vi "UHR-Fleezers Control (host) - Avogadro v3.vi"() -> ()   [LabVIEW 2014] (continued)
        n1387 = case shown="True" "Vortran Laser ON" {
          tunnel: "Laser interlacing mode" -> [_ w2246]
          tunnel: [enum32{"Laser ON", "Laser OFF", "Interlace"}."Laser OFF" ("Green laser mode") w2246] -> w2222
          tunnel: [FALSE w2242] -> w2221
          frame False {
          }
          frame True {
            n1388 = local read "Green FB On/Off"() -> (w2243:bool)
            n1389 = Equal?(x=w2246, y=enum32{"Laser ON", "Laser OFF", "Interlace"}."Interlace") -> (x = y?=w2244:bool)
            n1390 = And(x=w2244, y=w2243) -> (x .and. y?=w2242:bool)
          }
        }
        n1391 = case shown="True" "Red Laser ON" {
          tunnel: "Laser interlacing mode" -> [_ w2239]
          tunnel: [enum32{"Laser ON", "Laser OFF", "Interlace"}."Laser OFF" ("Green laser mode") w2239] -> w2218
          tunnel: [FALSE w2235] -> w2217
          frame False {
          }
          frame True {
            n1392 = local read "Red FB On/Off"() -> (w2236:bool)
            n1393 = Equal?(x=w2239, y=enum32{"Laser ON", "Laser OFF", "Interlace"}."Interlace") -> (x = y?=w2237:bool)
            n1394 = And(x=w2237, y=w2236) -> (x .and. y?=w2235:bool)
          }
        }
        n1395 = case shown="True" "Blue Laser ON" {
          tunnel: "Laser interlacing mode" -> [_ w2230]
          tunnel: [enum32{"Laser ON", "Laser OFF", "Interlace"}."Laser OFF" ("Green laser mode") w2230] -> w2214
          tunnel: [FALSE w2228] -> w2213
          frame False {
          }
          frame True {
            n1396 = local read "Blue FB On/Off"() -> (w2229:bool)
            n1397 = Equal?(x=w2230, y=enum32{"Laser ON", "Laser OFF", "Interlace"}."Interlace") -> (x = y?=w2231:bool)
            n1398 = And(x=w2231, y=w2229) -> (x .and. y?=w2228:bool)
          }
        }
        n1399 = xnode "Read/Write Control"("FPGA VI Reference In"=w2212, "Operating Mode"=w2222, "Operating Mode 2"=w2222, "Green FB On/Off"=w2221, "Red Laser Operating Mode"=w2218, "RI Operating Mode 2"=w2218, "Red FB On/Off"=w2217, "BI Operating Mode (AO)"=w2214, "Blue Laser Operating Mode (D)"=w2214, "Blue FB On/Off"=w2213) -> ("error out"=w2223:errorcluster)  [unwired: 1 in, 1 out]
        n1400 = local read "Red FB On/Off"() -> (w2195:bool)
        n1401 = local read "Vortran Laser ON"() -> (w2196:bool)
        n1402 = local read "Green FB On/Off"() -> (w2197:bool)
        n1403 = local read "Red Laser ON"() -> (w2194:bool)
        n1404 = And(x=w2195, y=w2194) -> (x .and. y?=w2200:bool)
        n1405 = And(x=w2197, y=w2196) -> (x .and. y?=w2206:bool)
        n1406 = local read "Red laser intensity (V)"() -> (w2199:dbl)
        n1407 = local read "Red FB Setpoint (mV)"() -> (w2198:dbl)
        n1408 = local read "Green FB Setpoint (mV)"() -> (w2209:dbl)
        n1409 = local read "Green laser intensity (V)"() -> (w2211:dbl)
        n1410 = Multiply(x=w2199, y=1000.0) -> (x*y=w2203:dbl)
        n1411 = Subtract(x=w2198, y=5.0) -> (x-y=w2202:dbl)
        n1412 = Multiply(x=w2211, y=1000.0) -> (x*y=w2208:dbl)
        n1413 = Subtract(x=w2209, y=5.0) -> (x-y=w2207:dbl)
        n1414 = Less Or Equal?(x=w2203, y=w2202) -> (x <= y?=w2201:bool)
        n1415 = Less Or Equal?(x=w2208, y=w2207) -> (x <= y?=w2205:bool)
        n1416 = And(x=w2200, y=w2201) -> (x .and. y?=w2190:bool)
        n1417 = And(x=w2206, y=w2205) -> (x .and. y?=w2191:bool)
        n1418 = Or(x=w2191, y=w2190) -> (x .or. y?=w2189:bool)
        n1419 = case shown="True" w2189 {
          frame False {
            n1420 = local write "Laser Intensity Low (bugs to fix)"(FALSE ("Laser Intensity Low")) -> ()
          }
          frame True {
            n1421 = local write "Laser Intensity Low (bugs to fix)"(TRUE ("Laser Intensity Low")) -> ()
          }
        }
      }
      event "Laser choice 0", "Laser choice 1", "Laser choice 2", "FL interlace ON count 0", "Fl interlace ON count 1", "FL interlace ON count 2", "FL interlace OFF count 0", "FL interlace OFF count 1", "FL interlace OFF count 2": Value Change {
        n1422 = event-data() -> ()  [unwired: 7 out]
        n1423 = xnode "Read/Write Control"("FPGA VI Reference In"=w2247, "FL interlace ON count 0"="FL interlace ON count 0", "Fl interlace ON count 1"="Fl interlace ON count 1", "FL interlace ON count 2"="FL interlace ON count 2", "FL interlace OFF count 0"="FL interlace OFF count 0", "FL interlace OFF count 1"="FL interlace OFF count 1", "FL interlace OFF count 2"="FL interlace OFF count 2", "Laser choice 0"="Laser choice 0", "Laser choice 1"="Laser choice 1", "Laser choice 2"="Laser choice 2") -> ()  [unwired: 1 in, 2 out]
      }
      event "Invert laser interlacing", "RF BD 2 to green AOM": Value Change {
        n1424 = event-data() -> ()  [unwired: 7 out]
        n1425 = local read "RF BD 2 to green AOM"() -> (w2257:bool)
        n1426 = xnode "Read/Write Control"("FPGA VI Reference In"=w2258, "Invert GI"="Invert laser interlacing", "Invert GI 2"="Invert laser interlacing", "Invert RI"="Invert laser interlacing", "Invert RI 2"="Invert laser interlacing", "Invert BI (AO)"="Invert laser interlacing", "Invert BI (D)"="Invert laser interlacing", "RF synth bd controls green"=w2257) -> ("error out"=w2260:errorcluster)  [unwired: 1 in, 1 out]
      }
      event "Green FB Setpoint (mV)", "Green FB Gains", "Green FB On/Off", "Green Intensity % (FB OFF)", "Green int current ON count adj": Value Change {
        n1427 = event-data() -> ()  [unwired: 7 out]
        n1428 = local read "Green FB Setpoint (mV)"() -> (w2280:dbl)
        n1429 = Multiply(x=w2280, y=3.2767) -> (x*y=w2279:dbl)
        n1430 = local read "Green Intensity % (FB OFF)"() -> (w2283:dbl)
        n1431 = Multiply(x=w2283, y=655.35) -> (x*y=w2284:dbl)
        n1432 = To Unsigned Word Integer(number=w2284) -> (unsigned 16bit integer=w2282:u16)
        n1433 = local read "Green int current ON count adj"() -> (w2286:u32)
        n1434 = local read "Laser interlacing mode"() -> (w2277:enum32{"Laser ON", "Laser OFF", "Interlace"})
        n1435 = local read "Green FB Gains"() -> (w2274:T18)
        n1436 = local read "Vortran Laser ON"() -> (w2278:bool)
        n1437 = local read "Green FB On/Off"() -> (w2287:bool)
        n1438 = Equal?(x=w2277, y=enum32{"Laser ON", "Laser OFF", "Interlace"}."Interlace") -> (x = y?=w2275:bool)
        n1439 = Unbundle By Name(w2274) -> ("proportional gain (Kc)"=w2273:i16, "integral gain (Kc*Ts/Ti)"=w2272:i16, "derivative gain (Kc*Td/Ts)"=w2271:i16)
        n1440 = Compound Arithmetic op=AND(w2275, w2287, w2278) -> (w2261:bool)
        n1441 = local read "Green FB Setpoint (mV)"() -> (w2265:dbl)
        n1442 = local read "Green laser intensity (V)"() -> (w2268:dbl)
        n1443 = xnode "Read/Write Control"("FPGA VI Reference In"=w2270, "Green FB Setpoint"=w2279, "Green FB On/Off"=w2261, "Current Out"=w2282, "Green int current ON count adj"=w2286, "P3"=w2273, "I3"=w2272, "D3"=w2271) -> ("error out"=w2288:errorcluster)  [unwired: 1 in, 1 out]
        n1444 = Multiply(x=w2268, y=1000.0) -> (x*y=w2264:dbl)
        n1445 = Subtract(x=w2265, y=5.0) -> (x-y=w2263:dbl)
        n1446 = Less Or Equal?(x=w2264, y=w2263) -> (x <= y?=w2262:bool)
        n1447 = And(x=w2261, y=w2262) -> (x .and. y?=w2269:bool)
        n1448 = case shown="True" w2269 {
          frame False {
            n1449 = local write "Laser Intensity Low (bugs to fix)"(FALSE ("Laser Intensity Low")) -> ()
          }
          frame True {
            n1450 = local write "Laser Intensity Low (bugs to fix)"(TRUE ("Laser Intensity Low")) -> ()
          }
        }
      }
      event "Blue FB Setpoint (mV)", "Blue FB Gains", "Blue FB On/Off", "Blue Intensity % (FB OFF)", "Blue int AO ON count adjust": Value Change {
        # "Triggers blue laser serial command"
        # "16 bit analog out"
        n1451 = event-data() -> ()  [unwired: 7 out]
        n1452 = Multiply(x="Blue FB Setpoint (mV)", y=3.2767) -> (x*y=w2308:dbl)
        n1453 = Multiply(x="Blue Intensity % (FB OFF)", y=0.8) -> (x*y=w2291:dbl)
        n1454 = Number To Decimal String(number=w2291) -> (decimal integer string=w2292:string)  [unwired: 1 in]
        n1455 = Multiply(x="Blue Intensity % (FB OFF)", y=655.35) -> (x*y=w2311:dbl)
        n1456 = local write "Blue Laser Power (mW)\n(Constant Power Mode)"(w2292) -> ()
        n1457 = To Unsigned Word Integer(number=w2311) -> (unsigned 16bit integer=w2310:u16)
        n1458 = local read "Laser interlacing mode"() -> (w2306:enum32{"Laser ON", "Laser OFF", "Interlace"})
        n1459 = Unbundle By Name("Blue FB Gains") -> ("proportional gain (Kc)"=w2303:i16, "integral gain (Kc*Ts/Ti)"=w2302:i16, "derivative gain (Kc*Td/Ts)"=w2301:i16)
        n1460 = local read "Blue Laser ON"() -> (w2296:bool)
        n1461 = Equal?(x=w2306, y=enum32{"Laser ON", "Laser OFF", "Interlace"}."Interlace") -> (x = y?=w2304:bool)
        n1462 = Compound Arithmetic op=AND(w2304, "Blue FB On/Off", w2296) -> (w2307:bool)
        n1463 = xnode "Read/Write Control"("FPGA VI Reference In"=w2295, "Blue FB Setpoint"=w2308, "Blue FB On/Off"=w2307, "BI Current Out"=w2310, "Blue current ON count adj (AO)"="Blue int AO ON count adjust", "P5"=w2303, "I5"=w2302, "D5"=w2301) -> ("error out"=w2313:errorcluster)  [unwired: 1 in, 1 out]
      }
      event "Red FB Setpoint (mV)", "Red FB Gains", "Red FB On/Off", "Red Intensity % (FB OFF)": Value Change {
        n1464 = event-data() -> ()  [unwired: 7 out]
        n1465 = local read "Red FB Setpoint (mV)"() -> (w2334:dbl)
        n1466 = Multiply(x=w2334, y=3.2767) -> (x*y=w2333:dbl)
        n1467 = local read "Red Intensity % (FB OFF)"() -> (w2324:dbl)
        n1468 = Multiply(x=w2324, y=655.35) -> (x*y=w2337:dbl)
        n1469 = To Unsigned Word Integer(number=w2337) -> (unsigned 16bit integer=w2336:u16)
        n1470 = local read "Laser interlacing mode"() -> (w2331:enum32{"Laser ON", "Laser OFF", "Interlace"})
        n1471 = local read "Red FB Gains"() -> (w2328:T18)
        n1472 = local read "Red Laser ON"() -> (w2332:bool)
        n1473 = local read "Red FB On/Off"() -> (w2339:bool)
        n1474 = Equal?(x=w2331, y=enum32{"Laser ON", "Laser OFF", "Interlace"}."Interlace") -> (x = y?=w2329:bool)
        n1475 = Unbundle By Name(w2328) -> ("proportional gain (Kc)"=w2327:i16, "integral gain (Kc*Ts/Ti)"=w2326:i16, "derivative gain (Kc*Td/Ts)"=w2325:i16)
        n1476 = Compound Arithmetic op=AND(w2329, w2339, w2332) -> (w2316:bool)
        n1477 = local read "Red laser intensity (V)"() -> (w2315:dbl)
        n1478 = local read "Red FB Setpoint (mV)"() -> (w2314:dbl)
        n1479 = xnode "Read/Write Control"("FPGA VI Reference In"=w2323, "Red FB Setpoint"=w2333, "Red FB On/Off"=w2316, "RI Current Out"=w2336, "P4"=w2327, "I4"=w2326, "D4"=w2325) -> ("error out"=w2340:errorcluster)  [unwired: 1 in, 1 out]
        n1480 = Multiply(x=w2315, y=1000.0) -> (x*y=w2320:dbl)
        n1481 = Subtract(x=w2314, y=5.0) -> (x-y=w2319:dbl)
        n1482 = Less Or Equal?(x=w2320, y=w2319) -> (x <= y?=w2318:bool)
        n1483 = And(x=w2316, y=w2318) -> (x .and. y?=w2317:bool)
        n1484 = case shown="False" w2317 {
          frame False {
            n1485 = local write "Laser Intensity Low (bugs to fix)"(FALSE ("Laser Intensity Low")) -> ()
          }
          frame True {
            n1486 = local write "Laser Intensity Low (bugs to fix)"(TRUE ("Laser Intensity Low")) -> ()
          }
        }
      }
      event "+ phase (APD 1 Gate)", "- phase (APD 1 Gate)", "+ phase (APD 2 Gate)", "- phase (APD 2 Gate)", "+ phase (APD 3 Gate)", "- phase (APD 3 Gate)", "+ phase (APD Acq)", "- phase (APD Acq)": Value Change {
        n1487 = event-data() -> ()  [unwired: 7 out]
        n1488 = local read "Phase Adj. (APD 1 Gate)"() -> (w2363:i16)
        n1489 = Or(x="- phase (APD 1 Gate)", y="+ phase (APD 1 Gate)") -> (x .or. y?=w2365:bool)
        n1490 = Negate(x=w2363) -> (-x=w2370:i16)
        n1491 = Select(t=w2370, s="+ phase (APD 1 Gate)", f=w2363) -> (s? t:f=w2369:i16)
        n1492 = local read "Phase Adj. (APD 2 Gate)"() -> (w2360:i16)
        n1493 = Or(x="- phase (APD 2 Gate)", y="+ phase (APD 2 Gate)") -> (x .or. y?=w2358:bool)
        n1494 = Negate(x=w2360) -> (-x=w2362:i16)
        n1495 = Select(t=w2362, s="+ phase (APD 2 Gate)", f=w2360) -> (s? t:f=w2359:i16)
        n1496 = Negate(x="Phase Adj. (APD 3 Gate)") -> (-x=w2357:i16)
        n1497 = Or(x="- phase (APD 3 Gate)", y="+ phase (APD 3 Gate)") -> (x .or. y?=w2353:bool)
        n1498 = Select(t=w2357, s="+ phase (APD 3 Gate)", f="Phase Adj. (APD 3 Gate)") -> (s? t:f=w2354:i16)
        n1499 = local read "Phase Adj. (APD Acq)"() -> (w2351:i16)
        n1500 = Or(x="- phase (APD Acq)", y="+ phase (APD Acq)") -> (x .or. y?=w2349:bool)
        n1501 = Negate(x=w2351) -> (-x=w2352:i16)
        n1502 = Select(t=w2352, s="+ phase (APD Acq)", f=w2351) -> (s? t:f=w2350:i16)
        n1503 = xnode "Read/Write Control"("FPGA VI Reference In"=w2343, "Phase count adjustment (APD 1 Gate)"=w2369, "Phase count adjustment (APD 2 Gate)"=w2359, "Phase count adjustment (APD 3 Gate)"=w2354, "Phase Count Adjustment (APD Acq)"=w2350) -> ("FPGA VI Reference Out"=w2367:T41, "error out"=w2368:errorcluster)  [unwired: 1 in]
        n1504 = xnode "Read/Write Control"("FPGA VI Reference In"=w2367, "error in"=w2368, "+ phase (APD 1 Gate)"=w2365, "+ phase (APD 2 Gate)"=w2358, "+ phase (APD 3 Gate)"=w2353, "+ phase (APD Acq)"=w2349) -> ("error out"=w2366:errorcluster)  [unwired: 1 out]
      }
      event "Invert APD Gate", "APD Gate ON Count", "APD Gate OFF Count", "APD Gate", "APD Integration Time (s)", "APD AO Scale Factor", "Duty Frequency (ON 1/N cycles)", "Interlace ON count", "Interlace OFF count": Value Change {
        n1505 = event-data() -> ()  [unwired: 7 out]
        n1506 = Add(x="Interlace ON count", y="Interlace OFF count") -> (x+y=w2377:u16)
        n1507 = Add(x="APD Gate ON Count", y="APD Gate OFF Count") -> (x+y=w2388:u16)
        n1508 = Multiply(x="Duty Frequency (ON 1/N cycles)", y=w2377) -> (x*y=w2373:u16)
        "Green AI Count" <- w2373
        "Red AI Count" <- w2373
        "Blue AI Count" <- w2373
        n1509 = Subtract(x=w2373, y="Interlace ON count") -> (x-y=w2376:u16)
        n1510 = Multiply(x=w2388, y="Duty Frequency (ON 1/N cycles)") -> (x*y=w2387:u16)
        n1511 = Subtract(x=w2387, y="APD Gate ON Count") -> (x-y=w2386:u16)
        n1512 = local read "DMA Update Period (s)"() -> (w2389:dbl)
        n1513 = Multiply(x="APD Integration Time (s)", y=40000000.0) -> (x*y=w2393:dbl)
        n1514 = Reciprocal(x="APD Integration Time (s)") -> (1/x=→"APD Acq Rate (Hz)":dbl)
        n1515 = To Unsigned Long Integer(number=w2393) -> (unsigned 32bit integer=w2379:u32)
        "APD Int. Count" <- w2379
        n1516 = local read "Number of APDs"() -> (w2372:u8)
        n1517 = Divide(x=w2389, y="APD Integration Time (s)") -> (x/y=w2391:dbl)
        n1518 = Multiply(x=w2372, y=w2391) -> (x*y=w2390:dbl)
        n1519 = local write "APD Samples/FIFO Acq."(w2391) -> ()
        n1520 = local write "APD Elements/DMA read"(w2390) -> ()
        n1521 = xnode "Read/Write Control"("FPGA VI Reference In"=w2371, "Invert APD Gate"="Invert APD Gate", "APD Gate ON Count"="APD Gate ON Count", "APD Gate OFF Count"=w2386, "APD Acq Rate Count"=w2379, "APD Gate Operating Mode"="APD Gate", "APD AO scale factor"="APD AO Scale Factor", "Green interlace ON count 2"="Interlace ON count", "Green interlace OFF count 2"=w2376, "Green FB Count"=w2373, "Red interlace ON count"="Interlace ON count", "Red interlace OFF count"="Interlace OFF count", "Blue ON count (AO)"="Interlace ON count", "Blue OFF count (AO)"="Interlace OFF count", "Blue interlace OFF count (D)"="Interlace OFF count", "Blue interlace ON count (D)"="Interlace ON count") -> ("error out"=w2395:errorcluster)  [unwired: 1 in, 1 out]
      }
      event "Neg. TTrig FPGA": Value Change {
        n1522 = event-data() -> ()  [unwired: 7 out]
        n1523 = xnode "Read/Write Control"("FPGA VI Reference In"=w2396, "TTrig Negate Pos"="Neg. TTrig FPGA") -> ()  [unwired: 1 in, 2 out]
      }
      event "Test ttrig": Value Change {
        n1524 = event-data() -> ()  [unwired: 7 out]
        n1525 = xnode "Read/Write Control"("FPGA VI Reference In"=w2398, "TTrig?"=TRUE) -> ("error out"=w2400:errorcluster)  [unwired: 1 in, 1 out]
      }
      event "Number of F/B Scans (AOD)", "Scan Speed (nm/s)", "Scan BD", "Initial delta (MHz)", "Step Size (nm)", "Scan Range (nm)": Value Change {
        w2464 = 123.0  # AOM cal (nm/MHz)
        n1526 = event-data() -> ()  [unwired: 7 out]
        n1527 = local read "BD 1 Frequency 1 (MHz)"() -> (w2447:dbl)
        n1528 = local read "AOM X Cal (nm/MHz)"() -> (w2439:dbl)
        n1529 = local read "X RF Frequency Limits (MHz)"() -> (w2451:T27)
        n1530 = local read "Y RF Frequency Limits (MHz)"() -> (w2448:T27)
        n1531 = local read "BD 2 Frequency 1 (MHz)"() -> (w2453:dbl)
        n1532 = Negate(x="Scan Range (nm)") -> (-x=w2417:dbl)
        n1533 = Divide(x=w2417, y=w2439) -> (x/y=w2421:dbl)
        n1534 = Select(t=w2451, s="Scan BD", f=w2448) -> (s? t:f=w2450:T27)
        n1535 = Select(t=w2447, s="Scan BD", f=w2453) -> (s? t:f=w2452:dbl)
        n1536 = Unbundle By Name(w2450) -> ("Maximum"=w2459:dbl, "Minimum"=w2458:dbl)
        n1537 = Add(x=w2421, y=w2452) -> (x+y=w2456:dbl)
        n1538 = Divide(x=w2417, y="Step Size (nm)") -> (x/y=w2436:dbl)
        n1539 = Divide(x="Step Size (nm)", y=w2439) -> (x/y=w2445:dbl)
        n1540 = Absolute Value(x=w2436) -> (abs(x)=w2420:dbl)
        n1541 = Sign(1:w2417) -> (0:w2418:dbl)
        n1542 = In Range and Coerce(upper limit=w2459, x=w2456, lower limit=w2458) -> (coerced(x)=w2455:dbl, In Range?=w2457:bool)
        n1543 = To Unsigned Quad Integer(1:w2420) -> (0:w2435:u64)
        "Scan steps (AOD)" <- w2435
        n1544 = call "IR AOM freq to word.vi"("Frequency In (MHz)"=w2445) -> ("Frequency Word Out (double)"=w2442:dbl)
        n1545 = Multiply(x=w2418, y=w2442) -> (x*y=w2419:dbl)
        n1546 = Subtract(x=w2456, y=w2455) -> (x-y=w2454:dbl)
        n1547 = To Quad Integer(1:w2419) -> (0:w2441:i64)
        "Incr. int (AOD)" <- w2441
        n1548 = Subtract(x=w2421, y=w2454) -> (x-y=w2440:dbl)
        "Scan Range (MHz)" <- w2440
        n1549 = Select(t=w2421, s=w2457, f=w2440) -> (s? t:f=w2460:dbl)
        n1550 = Multiply(x=w2440, y=w2439) -> (x*y=w2438:dbl)
        n1551 = Decrement(x=w2435) -> (x-1=w2488:u64)
        n1552 = Negate(x=w2438) -> (-x=w2434:dbl)
        n1553 = local write "Scan Range (nm)"(w2434) -> ()
        n1554 = Divide(x=w2460, y=w2488) -> (x/y=w2444:dbl)
        "Scan Increment (MHz)" <- w2444
        n1555 = call "IR AOM freq to word.vi"("Frequency In (MHz)"=w2444) -> ("Frequency Word Out (double)"=w2443:dbl)
        n1556 = Divide(x="Step Size (nm)", y="Scan Speed (nm/s)") -> (x/y=w2431:dbl)
        n1557 = To Quad Integer(1:w2443) -> ()  [unwired: 1 out]
        n1558 = local read "Number Interlace Sets"() -> (w2415:u8)
        n1559 = local read "AI Count (ticks)"() -> (w2416:u16)
        n1560 = local read "Total Counts (ticks)"() -> (w2414:u16)
        n1561 = local read "# Samples/trap"() -> (w2446:u32)
        n1562 = Multiply(x=w2416, y=w2415) -> (x*y=w2413:u16)
        n1563 = Divide(x=w2414, y=w2413) -> (x/y=w2412:dbl)
        n1564 = Select(t=w2447, s="Scan BD", f=w2453) -> (s? t:f=w2485:dbl)
        "Initial freq. (MHz)" <- w2485
        n1565 = Add(x=w2460, y=w2485) -> (x+y=→"Final freq. (MHz)":dbl)
        n1566 = Divide(x=w2414, y=40000000.0) -> (x/y=w2430:dbl)
        n1567 = Divide(x=w2431, y=w2430) -> (x/y=w2429:dbl)
        n1568 = To Unsigned Quad Integer(1:w2429) -> (0:w2404:u64)
        n1569 = Quotient & Remainder(x=w2404, y=u64 2) -> (x-y*floor(x/y)=w2408:u64)  [unwired: 1 out]
        n1570 = Equal?(x=w2408, y=u64 0) -> (x = y?=w2406:bool)
        n1571 = Decrement(x=w2404) -> (x-1=w2405:u64)
        n1572 = Select(t=w2404, s=w2406, f=w2405) -> (s? t:f=w2403:u64)
        "Cycles/step (AOD)" <- w2403
        n1573 = xnode "Read/Write Control"("FPGA VI Reference In"=w2402, "Scan steps"=w2435, "Number of scans"="Number of F/B Scans (AOD)", "Cycles per step"=w2403, "Scan freq.  increment"=w2441, "Scan BD"="Scan BD") -> ("error out"=w2494:errorcluster)  [unwired: 1 in, 1 out]
        n1574 = Multiply(x=w2435, y=w2403) -> (x*y=w2489:u64)
        n1575 = Multiply(x=w2489, y=u64 2) -> (x*y=w2411:u64)
        n1576 = Multiply(x=w2412, y=w2411) -> (x*y=w2410:dbl)
        "Data points/scan (f/b)" <- w2410
        n1577 = Multiply(x=w2410, y="Number of F/B Scans (AOD)") -> (x*y=w2492:dbl)
        "Data points/scans" <- w2492
        n1578 = Divide(x=w2492, y=w2446) -> (x/y=→"N sets should be saved":dbl)
        n1579 = Multiply(x=w2489, y=w2430) -> (x*y=w2428:dbl)
        "Time/Scan (s) (AOD)" <- w2428
        n1580 = Select(t=w2460, s="Scan BD", f=0.0) -> (s? t:f=w2486:dbl)
        n1581 = Select(t=0.0, s="Scan BD", f=w2460) -> (s? t:f=w2482:dbl)
        n1582 = local read "BD 2 Frequency 2 (MHz)"() -> (w2478:dbl)
        n1583 = local read "BD 1 Frequency 2 (MHz)"() -> (w2481:dbl)
        n1584 = Add(x=w2482, y=w2453) -> (x+y=w2479:dbl)
        n1585 = Add(x=w2447, y=w2486) -> (x+y=w2480:dbl)
        n1586 = Multiply(x=w2428, y=2.0) -> (x*y=w2427:dbl)
        n1587 = Multiply(x=w2427, y="Number of F/B Scans (AOD)") -> (x*y=w2424:dbl)
        n1588 = Divide(x=w2424, y=60.0) -> (x/y=→"Time to Finish All (min)":dbl)
        n1589 = Add(x="Trap 2 Bead Size (nm)", y="Trap 1 Bead Size (nm)") -> (x+y=w2468:dbl)
        n1590 = Divide(x=w2468, y=2.0) -> (x/y=w2462:dbl)
        n1591 = local read "Initial delta (MHz)"() -> (w2465:dbl)
        n1592 = Subtract(x=w2479, y=w2478) -> (x-y=w2476:dbl)
        n1593 = Subtract(x=w2480, y=w2481) -> (x-y=w2477:dbl)
        n1594 = Square(x=w2476) -> (x^2=w2475:dbl)
        n1595 = Square(x=w2477) -> (x^2=w2474:dbl)
        n1596 = Add(x=w2474, y=w2475) -> (x+y=w2473:dbl)
        n1597 = Square Root(x=w2473) -> (sqrt(x)=w2472:dbl)
        "Final delta (MHz)" <- w2472
        n1598 = Multiply(x=w2464, y=w2472) -> (x*y=w2471:dbl)
        n1599 = Multiply(x=w2465, y=w2464) -> (x*y=w2463:dbl)
        n1600 = Subtract(x=w2463, y=w2462) -> (x-y=→"Initial sep (nm)":dbl)
        n1601 = Subtract(x=w2471, y=w2462) -> (x-y=→"Final sep (nm)":dbl)
      }
      event "Swap F1 and F2", "RF amplitude switch delay": Value Change {
        n1602 = event-data() -> ()  [unwired: 7 out]
        n1603 = local read "RF amplitude switch delay"() -> (w2496:u16)
        n1604 = local read "Swap F1 and F2"() -> (w2497:bool)
        n1605 = xnode "Read/Write Control"("FPGA VI Reference In"=w2495, "Swap F1 and F2"=w2497, "Amp switch delay"=w2496) -> ("error out"=w2498:errorcluster)  [unwired: 1 in, 1 out]
      }
      event "Scan steps (MCL)", "Number of scans (MCL)", "Scan Range (V)\n(of steps)", "2D or 1D Scan", "N APD Samp/step", "Fast Scan Dir", "Continuous MCL Scanning", "Scan lines (y)": Value Change {
        w2501 = 32767.0 ("y")
        n1606 = event-data() -> ()  [unwired: 7 out]
        n1607 = Select(t="Scan lines (y)", s="2D or 1D Scan", f="Number of scans (MCL)") -> (s? t:f=w2506:u64)
        n1608 = Decrement(x="Scan steps (MCL)") -> (x-1=w2522:u64)
        n1609 = Divide(x="Scan Range (V)\n(of steps)", y=w2522) -> (x/y=w2521:dbl)
        "Desired Scan Incr (V)" <- w2521
        n1610 = local read "APD Integration Time (s)"() -> (w2514:dbl)
        n1611 = Multiply(x=w2521, y=w2501) -> (x*y=w2530:dbl)
        n1612 = Divide(x=w2530, y=10.0) -> (x/y=w2520:dbl)
        "Desired incr (int)" <- w2520
        n1613 = local read "Update Count (MCL)"() -> (w2526:u32)
        n1614 = Round Toward -Infinity(1:w2520) -> (0:w2529:dbl)
        n1615 = To Word Integer(number=w2529) -> (16bit integer=w2504:i16)
        "Actual Incr. int (MCL)" <- w2504
        n1616 = Multiply(x=w2514, y=40000000.0) -> (x*y=w2527:dbl)
        n1617 = Divide(x=w2527, y=w2526) -> (x/y=w2525:dbl)
        n1618 = Multiply(x=i16 10, y=w2504) -> (x*y=w2502:i16)
        n1619 = Multiply(x="N APD Samp/step", y=w2525) -> (x*y=w2524:dbl)
        "Cycles/step (MCL)" <- w2524
        n1620 = Divide(x=w2502, y=w2501) -> (x/y=→"Actual MCL Inc (V)":dbl)
        n1621 = Multiply(x="N APD Samp/step", y="Scan steps (MCL)") -> (x*y=w2516:dbl)
        n1622 = local read "APD Samples/FIFO Acq."() -> (w2513:dbl)
        n1623 = Multiply(x=w2516, y=u64 2) -> (x*y=w2515:dbl)
        "Data points/scan (f+b)" <- w2515
        n1624 = Multiply(x=w2515, y=w2506) -> (x*y=w2533:dbl)
        "Data points/scans (MCL)" <- w2533
        n1625 = Multiply(x=w2514, y=w2515) -> (x*y=w2507:dbl)
        "Time/f+b scan (s) (MCL)" <- w2507
        n1626 = Divide(x=w2533, y=w2513) -> (x/y=→"N sets should be saved (MCL)":dbl)
        n1627 = Multiply(x=w2507, y=w2506) -> (x*y=→"Total Time (s)":dbl)
        n1628 = Not(x="Fast Scan Dir") -> (.not. x?=w2511:bool)
        n1629 = xnode "Read/Write Control"("FPGA VI Reference In"=w2499, "Scan steps (MCL)"="Scan steps (MCL)", "Number of scans (MCL)"=w2506, "Cycles per step (MCL)"=w2524, "Scan freq.  increment (MCL)"=w2504, "1D or 2D Scan?"="2D or 1D Scan", "MCL Scan Axis"=w2511, "Cont. Scan (MCL)"="Continuous MCL Scanning") -> ("error out"=w2535:errorcluster)  [unwired: 1 in, 1 out]
      }
      event "Read Cal": Value Change {
        w2558 = T54."big-endian, network order" ("byte order (0:big-endian, network order)")
        n1630 = event-data() -> ()  [unwired: 7 out]
        n1631 = local read "Save file name"() -> (w2583:path)
        n1632 = Strip Path(path=w2583) -> (stripped path=w2582:path)  [unwired: 1 out]
        n1633 = Path To String(path=w2582) -> (string=w2575:string)
        n1634 = Concatenate Strings(w2575, "\\current.cal" ("string")) -> (w2580:string)
        n1635 = String To Path(string=w2580) -> (path=w2579:path)
        n1636 = Concatenate Strings(w2575, "\\current.off" ("string")) -> (w2573:string)
        n1637 = Open/Create/Replace File(file path (use dialog)=w2579, operation (0:open)=T53."open", access (0:read/write)=enum16{"read/write", "read-only", "write-only"}."read-only") -> (refnum out=w2586:refnum<file>, error out=w2578:errorcluster)  [unwired: 1 in, 3 out]
        n1638 = Deny Access(4:w2578, 7:w2586) -> (0:w2559:errorcluster, 3:w2554:refnum<file>)  [unwired: 1 out]
        n1639 = String To Path(string=w2573) -> (path=w2570:path)
        n1640 = local write "Read Cal"(FALSE ("Read Cal")) -> ()
        n1641 = Open/Create/Replace File(file path (use dialog)=w2570, operation (0:open)=T53."open", access (0:read/write)=enum16{"read/write", "read-only", "write-only"}."read-only") -> (refnum out=w2569:refnum<file>)  [unwired: 1 in, 4 out]
        n1642 = Deny Access(7:w2569) -> (3:w2568:refnum<file>)  [unwired: 1 in, 2 out]
        n1643 = Read from Binary File(5:0.0, 9:w2558, 10:-1 ("count (1)"), 11:w2568) -> (2:w2536:dbl[], 3:w2565:refnum<file>)  [unwired: 1 in, 3 out]
        "Raw offsets" <- w2536
        n1644 = local read "Multiple-MCL offset?"() -> (w2537:bool)
        n1645 = Close File(refnum=w2565) -> ()  [unwired: 1 in, 2 out]
        n1646 = case shown="True" w2537 {
          tunnel: w2536 -> [w2591 w2598]
          tunnel: [w2588 w2596] -> w2563
          tunnel: [w2587 w2595] -> w2562
          frame False {
            # "If not doing multiple offset, same calculation as before"
            n1647 = Decimate 1D Array(w2591) -> (w2588:dbl[], w2587:dbl[])
            n1648 = Bundle By Name(cluster="Two Trap Offset Values", "Trap 1X offset"=w2588, "Trap 2X offset"=w2587) -> (w2589:T32)
            n1649 = local write "Two Trap Offset Values"(w2589) -> ()
          }
          frame True {
            w2593 = 0.0
            # "When doing multiple offset: separate data to different scans, make array of clusters of 1x,1y,2x,2y,3x,3y arrays"
            n1650 = local read "MCL offset scanning range (V)"() -> (w2599:T4)
            n1651 = local read "Offset file step size"() -> (w2597:dbl)
            n1652 = Build Array(w2593, w2593, w2593, w2593, w2593, w2593) -> (w2592:dbl[])
            n1653 = call "generate multiple MCL offset.vi"("Offset array"=w2598, "offset file step size"=w2597, "MCL offset scanning range (V)"=w2599, "Corrections"=w2592) -> ("B_X mean out"=w2595:dbl[], "A_X mean out"=w2596:dbl[], "Output array"=→"Multi-MCL offset array":T31)
          }
        }
        n1654 = Build Array("T1 calibration", "T2 calibration", "T3 calibration") -> (w2550:T56)
        n1655 = for {
          N: 3 ("count (1)") -> [_]
          tunnel: w2558 -> [w2617]
          shift-right: [w2615] -> w2556
          shift-left: w2559 -> [w2618]
          shift-right: [w2614] -> w2555
          shift-left: w2554 -> [w2613]
          tunnel: w2550 -> [w2612] mode=indexing
          tunnel: [w2606] -> w2549 mode=indexing
          i -> [w2607]
          w2601 = 1000.0
          n1656 = Read from Binary File(5:0.0, 8:w2618, 9:w2617, 10:6 ("count (1)"), 11:w2613) -> (0:w2615:errorcluster, 2:w2620:dbl[], 3:w2614:refnum<file>)  [unwired: 2 out]
          n1657 = Array To Cluster(array=w2620) -> (cluster=w2611:T57)
          n1658 = Unbundle(w2611) -> ("[0]"=w2610:dbl, "[1]"=w2609:dbl, "[2]"=w2603:dbl, "[3]"=w2608:dbl, "[4]"=w2602:dbl, "[5]"=w2605:dbl)
          n1659 = Multiply(x=w2602, y=w2601) -> (x*y=w2600:dbl)
          n1660 = Multiply(x=w2601, y=w2605) -> (x*y=w2604:dbl)
          n1661 = Bundle By Name(cluster=w2612, "alpha_x (nm/V)"=w2610, "alpha_y (nm/V)"=w2609, "kappa_x (pN/nm)"=w2603, "kappa_y (pN/nm)"=w2608, "offset_x (mV)"=w2600, "offset_y (mV)"=w2604) -> (w2606:T12)
          n1662 = case shown="2" w2607 {
            tunnel: w2606 -> [w2621 w2622 w2623]
            frame 0, Default {
              n1663 = local write "T1 calibration"(w2621) -> ()
            }
            frame 1 {
              n1664 = local write "T2 calibration"(w2622) -> ()
            }
            frame 2 {
              n1665 = local write "T3 calibration"(w2623) -> ()
            }
          }
        }
        n1666 = Index Array(array=w2549, index=1) -> (element=w2546:T12)
        n1667 = Index Array(array=w2549, index=0) -> (element=w2545:T12)
        n1668 = Unbundle By Name(w2546) -> ("alpha_x (nm/V)"=w2544:dbl, "kappa_x (pN/nm)"=w2543:dbl)
        n1669 = Unbundle By Name(w2545) -> ("alpha_x (nm/V)"=w2542:dbl, "kappa_x (pN/nm)"=w2541:dbl)
        n1670 = Close File(refnum=w2555, error in=w2556) -> (error out=→"Read cal error":errorcluster)  [unwired: 1 out]
        n1671 = Multiply(x=w2544, y=w2543) -> (x*y=w2540:dbl)
        n1672 = Multiply(x=w2542, y=w2541) -> (x*y=w2539:dbl)
        n1673 = Divide(x=w2540, y=w2539) -> (x/y=w2538:dbl)
        n1674 = property on="B factor" class="DigNum (strict)"("Val(Sgnl)"=w2538) -> ()  [unwired: 2 in, 2 out]
        n1675 = Multiply(x=w2562, y=w2538) -> (x*y=w2564:dbl[])
        n1676 = Subtract(x=w2563, y=w2564) -> (x-y=w2560:dbl[])
        n1677 = case shown="True" "Auto read offset correction" {
          tunnel: w2560 -> [_ w2624]
          frame False {
          }
          frame True {
            n1678 = property on="Setpoint offset\ncorrection values" class="Arr (strict)"("Val(Sgnl)"=w2624) -> ()  [unwired: 2 in, 2 out]
          }
        }
      }
      event "Abort MCL Scan": Value Change {
        n1679 = event-data() -> ()  [unwired: 7 out]
        n1680 = local write "MCL Scanning"(FALSE ("MCL Scanning")) -> ()
        n1681 = xnode "Read/Write Control"("FPGA VI Reference In"=w2625, "Abort scan (MCL)"="Abort MCL Scan") -> ("error out"=w2628:errorcluster)  [unwired: 1 in, 1 out]
      }
      event "Update Count (MCL)": Value Change {
        n1682 = event-data() -> ()  [unwired: 7 out]
        n1683 = xnode "Read/Write Control"("FPGA VI Reference In"=w2629, "MCL count"="Update Count (MCL)") -> ("error out"=w2631:errorcluster)  [unwired: 1 in, 1 out]
      }
      event "+ phase (MCL)", "- phase (MCL)": Value Change {
        n1684 = event-data() -> ()  [unwired: 7 out]
        n1685 = Or(x="- phase (MCL)", y="+ phase (MCL)") -> (x .or. y?=w2635:bool)
        n1686 = Negate(x="Phase adjust (MCL)") -> (-x=w2641:i16)
        n1687 = Select(t=w2641, s="+ phase (MCL)", f="Phase adjust (MCL)") -> (s? t:f=w2639:i16)
        n1688 = xnode "Read/Write Control"("FPGA VI Reference In"=w2632, "Phase count adjustment (MCL)"=w2639) -> ("FPGA VI Reference Out"=w2636:T41, "error out"=w2637:errorcluster)  [unwired: 1 in]
        n1689 = xnode "Read/Write Control"("FPGA VI Reference In"=w2636, "error in"=w2637, "+ phase (MCL)"=w2635) -> ("error out"=w2634:errorcluster)  [unwired: 1 out]
      }
      event "Abort AOD Scan": Value Change {
        n1690 = event-data() -> ()  [unwired: 7 out]
        n1691 = xnode "Read/Write Control"("FPGA VI Reference In"=w2642, "Abort scan"="Abort AOD Scan") -> ("error out"=w2644:errorcluster)  [unwired: 1 in, 1 out]
      }
      event "Continuous AOD Scanning": Value Change {
        n1692 = event-data() -> ()  [unwired: 7 out]
        n1693 = xnode "Read/Write Control"("FPGA VI Reference In"=w2645, "Cont. Scan"="Continuous AOD Scanning") -> ("error out"=w2647:errorcluster)  [unwired: 1 in, 1 out]
      }
      event "Index": Value Change {
        n1694 = event-data() -> ()  [unwired: 7 out]
        n1695 = call "Create new save file.vi"("Insert"="", "Ext"=".dat" ("string"), "Index In"="Index") -> ("Path Out"=→"Save file name":path, "Index Out"=w2648:dbl)
        "Save index" <- w2648
        n1696 = local write "Index"(w2648) -> ()
      }
      event "AO1", "AO2": Value Change {
        w2662 = 10.0 ("y")
        w2661 = 32767.0 ("y")
        n1697 = event-data() -> ()  [unwired: 7 out]
        n1698 = local read "AO2"() -> (w2660:dbl)
        n1699 = local read "AO1"() -> (w2657:dbl)
        n1700 = Multiply(x=w2657, y=w2661) -> (x*y=w2656:dbl)
        n1701 = Multiply(x=w2660, y=w2661) -> (x*y=w2659:dbl)
        n1702 = Divide(x=w2656, y=w2662) -> (x/y=w2655:dbl)
        n1703 = Divide(x=w2659, y=w2662) -> (x/y=w2658:dbl)
        n1704 = To Word Integer(number=w2655) -> (16bit integer=w2663:i16)
        n1705 = To Word Integer(number=w2658) -> (16bit integer=w2664:i16)
        n1706 = xnode "Read/Write Control"("FPGA VI Reference In"=w2653, "AO1 (Y)"=w2663, "AO2 (X)"=w2664) -> ("error out"=w2654:errorcluster)  [unwired: 1 in, 1 out]
      }
      event "Inject Pump 1": Value Change {
        n1707 = event-data() -> ()  [unwired: 7 out]
        n1708 = disable-structure shown="Disabled" {
          disable-tunnel: w2665 -> [w2666 _]
          frame Disabled {
            n1709 = local read "Use Harvard pumps\nfor beads (else Chemyx)"() -> (w2667:bool)
            n1710 = case shown="True" w2667 {
              tunnel: "Inject Pump 1" -> [w2671 w2712]
              tunnel: w2666 -> [_ w2713]
              frame False {
                n1711 = local read "Pump write delay (ms)"() -> (w2670:dbl)
                n1712 = local read "Chemyx Syringe Pump Serial Port"() -> (w2669:refnum<visa-resource-name>)
                n1713 = case shown="True" w2671 {
                  tunnel: w2670 -> [w2677 w2691]
                  tunnel: w2669 -> [w2674 w2690]
                  frame False {
                    n1714 = flat-sequence {
                      tunnel: w2674 -> [w2678]
                      tunnel: [w2678] -> w2675
                      tunnel: w2677 -> [_]
                      tunnel: [w2681] -> w2676
                      tunnel: w2675 -> [w2681]
                      tunnel: w2676 -> [w2682]
                      tunnel: [w2682] -> w2672
                      tunnel: [w2684] -> w2673
                      tunnel: w2672 -> [w2684]
                      tunnel: w2673 -> [w2686]
                      frame #0 {
                        n1715 = call "Write to pump.vi"("string"="enter pump1", "VISA resource name"=w2678) -> ()  [unwired: 1 out]
                      }
                      frame #1 {
                        n1716 = Wait (ms)(milliseconds to wait="Pump pause delay (ms)") -> ()  [unwired: 1 out]
                      }
                      frame #2 {
                        n1717 = call "Write to pump.vi"("string"="stop", "VISA resource name"=w2682) -> ()  [unwired: 1 out]
                      }
                      frame #3 {
                        n1718 = Wait (ms)(milliseconds to wait=u32 500) -> ()  [unwired: 1 out]
                      }
                      frame #4 {
                        n1719 = call "Write to pump.vi"("string"="stop", "VISA resource name"=w2686) -> ()  [unwired: 1 out]
                      }
                    }
                  }
                  frame True {
                    n1720 = flat-sequence {
                      tunnel: w2690 -> [w2700]
                      tunnel: w2691 -> [w2695]
                      tunnel: w2691 -> [w2702]
                      tunnel: w2690 -> [w2703]
                      tunnel: [w2703] -> w2688
                      tunnel: [w2705] -> w2689
                      tunnel: w2688 -> [w2705]
                      tunnel: w2689 -> [w2707]
                      frame #0 {
                        n1721 = local read "All Pump Parameters"() -> (w2694:T14)
                        n1722 = Unbundle By Name(w2694) -> ("Pump 1"=w2701:T58)
                        n1723 = call "Set pump parameters.vi"("Pump write delay (ms)"=w2695, "Volume (uL)"="Ch 1 Inject Volume (uL)", "Rate (uL/h)"="Ch 1 Inject Rate (ul/h)", "Units"=4.0, "Pump #"=1.0, "Pump Parameters In"=w2701, "VISA resource name"=w2700) -> ("Pump Parameters Out"=w2693:T58)  [unwired: 3 in]
                        n1724 = Bundle By Name(cluster=w2694, "Pump 1"=w2693) -> (w2692:T14)
                        n1725 = local write "All Pump Parameters"(w2692) -> ()
                      }
                      frame #1 {
                        n1726 = Wait (ms)(milliseconds to wait=w2702) -> ()  [unwired: 1 out]
                      }
                      frame #2 {
                        n1727 = call "Write to pump.vi"("string"="start", "VISA resource name"=w2703) -> ()  [unwired: 1 out]
                      }
                      frame #3 {
                        n1728 = Wait (ms)(milliseconds to wait=u32 500) -> ()  [unwired: 1 out]
                      }
                      frame #4 {
                        n1729 = call "Write to pump.vi"("string"="start", "VISA resource name"=w2707) -> ()  [unwired: 1 out]
                      }
                    }
                  }
                }
              }
              frame True {
                n1730 = case shown="False" w2712 {
                  tunnel: w2713 -> [w2725 w2735]
                  frame False {
                    n1731 = flat-sequence {
                      tunnel: w2725 -> [w2727]
                      frame #0 {
                        n1732 = local write "Flushing P1"(FALSE ("Flushing P1")) -> ()
                        n1733 = Concatenate Strings("stop" ("string"), "\r") -> (w2729:string)
                        n1734 = VISA Write(VISA resource name=w2727, write buffer=w2729) -> ()  [unwired: 1 in, 3 out]
                      }
                      frame #1 {
                        n1735 = property on="Clear Volume P1" class="Bool (strict)"("Val(Sgnl)"=TRUE ("Value (Signaling)")) -> ()  [unwired: 2 in, 2 out]
                      }
                    }
                  }
                  frame True {
                    n1736 = local read "Normal Flow Rate (ul/h) P1"() -> (w2733:dbl)
                    n1737 = Number To Decimal String(number=w2733) -> (decimal integer string=w2739:string)  [unwired: 1 in]
                    n1738 = Concatenate Strings("irate  " ("string"), w2739, " u/h" ("string"), "\r") -> (w2737:string)
                    n1739 = VISA Write(VISA resource name=w2735, write buffer=w2737) -> (VISA resource name out=w2734:refnum<visa-resource-name>)  [unwired: 1 in, 2 out]
                    n1740 = Concatenate Strings("irun" ("string"), "\r") -> (w2741:string)
                    n1741 = VISA Write(VISA resource name=w2734, write buffer=w2741) -> ()  [unwired: 1 in, 3 out]
                  }
                }
                n1742 = local read "Saving..."() -> (w2710:bool)
                n1743 = local read "Save Event Log?"() -> (w2709:bool)
                n1744 = And(x=w2710, y=w2709) -> (x .and. y?=w2711:bool)
                n1745 = case shown="True" w2711 {
                  tunnel: w2712 -> [_ w2723]
                  frame False {
                  }
                  frame True {
                    n1746 = local read "Normal Flow Rate (ul/h) P1"() -> (w2714:dbl)
                    n1747 = Number To Decimal String(number=w2714) -> (decimal integer string=w2715:string)  [unwired: 1 in]
                    n1748 = Concatenate Strings("on, flow rate", w2715) -> (w2717:string)
                    n1749 = Select(t=w2717, s=w2723, f="off") -> (s? t:f=w2719:string)
                    n1750 = local read "log file ref"() -> (w2724:refnum<file>)
                    n1751 = local read "Time (s)"() -> (w2718:dbl)
                    n1752 = Concatenate Strings("pump 1 ", w2719) -> (w2721:string)
                    n1753 = call "write to event log.vi"("log file ref"=w2724, "time"=w2718, "input string"=w2721) -> ()  [unwired: 8 in]
                  }
                }
              }
            }
          }
          frame Enabled {
          }
        }
      }
      event "Shunt 1": Value Change {
        n1754 = event-data() -> ()  [unwired: 7 out]
        n1755 = local read "Visa resource for valves"() -> (w2743:refnum<visa-resource-name>)
        n1756 = call "hamilton_controller.vi"("VISA resource name in"=w2743, "Open?"="Shunt 1", "valve"=enum16{"A", "B", "ALL"}."A", "action"=T49."MOVE VALVE") -> ("error out"=w2745:errorcluster)  [unwired: 6 in, 1 out]
      }
      event "Shunt 2": Value Change {
        n1757 = event-data() -> ()  [unwired: 7 out]
        n1758 = case shown="True" "Shunt 2" {
          tunnel: [w2752 w2758] -> w2750
          tunnel: w2748 -> [_ w2756]
          frame False {
            n1759 = local read "Visa resource for valves"() -> (w2753:refnum<visa-resource-name>)
            n1760 = call "hamilton_controller.vi"("VISA resource name in"=w2753, "Open?"=FALSE, "valve"=enum16{"A", "B", "ALL"}."B", "action"=T49."MOVE VALVE") -> ("error out"=w2752:errorcluster)  [unwired: 6 in, 1 out]
          }
          frame True {
            n1761 = case shown="True" "Auto switch off shunt?" {
              tunnel: [w2761 w2772] -> w2758
              tunnel: w2756 -> [_ w2765]
              frame False {
                n1762 = local read "Visa resource for valves"() -> (w2760:refnum<visa-resource-name>)
                n1763 = call "hamilton_controller.vi"("VISA resource name in"=w2760, "Open?"=TRUE, "valve"=enum16{"A", "B", "ALL"}."B", "action"=T49."MOVE VALVE") -> ("error out"=w2761:errorcluster)  [unwired: 6 in, 1 out]
              }
              frame True {
                n1764 = flat-sequence {
                  tunnel: [w2776] -> w2773
                  tunnel: [w2775] -> w2766
                  tunnel: w2765 -> [w2775]
                  tunnel: [w2782] -> w2774
                  tunnel: w2773 -> [w2782]
                  tunnel: [w2781] -> w2767
                  tunnel: w2766 -> [w2781]
                  tunnel: w2774 -> [w2788]
                  tunnel: [w2787] -> w2770
                  tunnel: [w2786] -> w2768
                  tunnel: w2767 -> [w2786]
                  tunnel: [w2794] -> w2771
                  tunnel: w2770 -> [w2794]
                  tunnel: [w2793] -> w2769
                  tunnel: w2768 -> [w2793]
                  tunnel: w2771 -> [w2797]
                  tunnel: w2769 -> [w2796]
                  tunnel: [w2797] -> w2764
                  tunnel: [w2802] -> w2772
                  tunnel: w2764 -> [w2802]
                  frame #0 {
                    n1765 = local read "Visa resource for valves"() -> (w2778:refnum<visa-resource-name>)
                    n1766 = call "hamilton_controller.vi"("VISA resource name in"=w2778, "Open?"=TRUE, "valve"=enum16{"A", "B", "ALL"}."B", "action"=T49."MOVE VALVE") -> ("error out"=w2776:errorcluster)  [unwired: 6 in, 1 out]
                  }
                  frame #1 {
                    n1767 = Multiply(x="Shunt switch off time (s)", y=1000) -> (x*y=w2783:i32)
                    n1768 = Wait (ms)(milliseconds to wait=w2783) -> ()  [unwired: 1 out]
                  }
                  frame #2 {
                    n1769 = local read "Visa resource for valves"() -> (w2791:refnum<visa-resource-name>)
                    n1770 = call "hamilton_controller.vi"("VISA resource name in"=w2791, "error in"=w2788, "Open?"=FALSE, "valve"=enum16{"A", "B", "ALL"}."B", "action"=T49."MOVE VALVE") -> ("error out"=w2787:errorcluster)  [unwired: 5 in, 1 out]
                  }
                  frame #3 {
                    n1771 = Wait (ms)(milliseconds to wait=1000) -> ()  [unwired: 1 out]
                  }
                  frame #4 {
                    n1772 = case shown="True" "Force FB at end of shunt?" {
                      tunnel: w2796 -> [_ w2800]
                      frame False {
                      }
                      frame True {
                        w2799 = TRUE
                        n1773 = local write "Trap Pos. FB ON"(w2799) -> ()
                        n1774 = xnode "Read/Write Control"("FPGA VI Reference In"=w2800, "Force feedback"=w2799) -> ()  [unwired: 1 in, 2 out]
                      }
                    }
                  }
                  frame #5 {
                    n1775 = local write "Shunt 2"(FALSE) -> ()
                  }
                }
              }
            }
          }
        }
      }
      event "Inject Pump 3": Value Change {
        n1776 = event-data() -> ()  [unwired: 7 out]
        n1777 = local read "Use Harvard pumps\nfor beads (else Chemyx)"() -> (w2804:bool)
        n1778 = disable-structure shown="Disabled" {
          disable-tunnel: w2804 -> [w2806 _]
          disable-tunnel: w2803 -> [w2805 _]
          frame Disabled {
            n1779 = case shown="True" w2806 {
              tunnel: "Inject Pump 3" -> [w2810 w2851]
              tunnel: w2805 -> [_ w2852]
              frame False {
                n1780 = local read "Pump write delay (ms)"() -> (w2809:dbl)
                n1781 = case shown="True" w2810 {
                  tunnel: w2809 -> [w2816 w2830]
                  tunnel: "Chemyx Syringe Pump Serial Port" -> [w2813 w2829]
                  frame False {
                    n1782 = flat-sequence {
                      tunnel: w2813 -> [w2817]
                      tunnel: [w2817] -> w2814
                      tunnel: w2816 -> [_]
                      tunnel: [w2820] -> w2815
                      tunnel: w2814 -> [w2820]
                      tunnel: w2815 -> [w2821]
                      tunnel: [w2821] -> w2811
                      tunnel: [w2823] -> w2812
                      tunnel: w2811 -> [w2823]
                      tunnel: w2812 -> [w2825]
                      frame #0 {
                        n1783 = call "Write to pump.vi"("string"="enter pump3", "VISA resource name"=w2817) -> ()  [unwired: 1 out]
                      }
                      frame #1 {
                        n1784 = local read "Pump pause delay (ms)"() -> (w2819:u32)
                        n1785 = Wait (ms)(milliseconds to wait=w2819) -> ()  [unwired: 1 out]
                      }
                      frame #2 {
                        n1786 = call "Write to pump.vi"("string"="stop", "VISA resource name"=w2821) -> ()  [unwired: 1 out]
                      }
                      frame #3 {
                        n1787 = Wait (ms)(milliseconds to wait=u32 0) -> ()  [unwired: 1 out]
                      }
                      frame #4 {
                        n1788 = call "Write to pump.vi"("string"="stop", "VISA resource name"=w2825) -> ()  [unwired: 1 out]
                      }
                    }
                  }
                  frame True {
                    n1789 = flat-sequence {
                      tunnel: w2829 -> [w2839]
                      tunnel: w2830 -> [w2834]
                      tunnel: w2830 -> [w2841]
                      tunnel: w2829 -> [w2842]
                      tunnel: [w2842] -> w2828
                      tunnel: [w2845] -> w2827
                      tunnel: w2828 -> [w2845]
                      tunnel: w2827 -> [w2846]
                      frame #0 {
                        n1790 = local read "All Pump Parameters"() -> (w2833:T14)
                        n1791 = Unbundle By Name(w2833) -> ("Pump 3"=w2840:T58)
                        n1792 = call "Set pump parameters.vi"("Pump write delay (ms)"=w2834, "Volume (uL)"="Ch 3 Inject Volume (uL)", "Rate (uL/h)"="Ch 3 Inject Rate (ul/h)", "Units"=4.0, "Pump #"=3.0, "Pump Parameters In"=w2840, "VISA resource name"=w2839) -> ("Pump Parameters Out"=w2832:T58)  [unwired: 3 in]
                        n1793 = Bundle By Name(cluster=w2833, "Pump 3"=w2832) -> (w2831:T14)
                        n1794 = local write "All Pump Parameters"(w2831) -> ()
                      }
                      frame #1 {
                        n1795 = Wait (ms)(milliseconds to wait=w2841) -> ()  [unwired: 1 out]
                      }
                      frame #2 {
                        n1796 = call "Write to pump.vi"("string"="start", "VISA resource name"=w2842) -> ()  [unwired: 1 out]
                      }
                      frame #3 {
                        n1797 = Wait (ms)(milliseconds to wait=u32 500) -> ()  [unwired: 1 out]
                      }
                      frame #4 {
                        n1798 = call "Write to pump.vi"("string"="start", "VISA resource name"=w2846) -> ()  [unwired: 1 out]
                      }
                    }
                  }
                }
              }
              frame True {
                n1799 = case shown="False" w2851 {
                  tunnel: w2852 -> [w2864 w2871]
                  frame False {
                    n1800 = flat-sequence {
                      tunnel: w2864 -> [w2866]
                      frame #0 {
                        n1801 = local write "Flushing P3"(FALSE ("Flushing P3")) -> ()
                        n1802 = Concatenate Strings("stop" ("string"), "\r") -> (w2868:string)
                        n1803 = VISA Write(VISA resource name=w2866, write buffer=w2868) -> ()  [unwired: 1 in, 3 out]
                      }
                      frame #1 {
                        n1804 = property on="Clear Volume P3" class="Bool (strict)"("Val(Sgnl)"=TRUE ("Value (Signaling)")) -> ()  [unwired: 2 in, 2 out]
                      }
                    }
                  }
                  frame True {
                    n1805 = local read "Normal Flow Rate (ul/h) P3"() -> (w2872:dbl)
                    n1806 = Number To Decimal String(number=w2872) -> (decimal integer string=w2878:string)  [unwired: 1 in]
                    n1807 = Concatenate Strings("irate  " ("string"), w2878, " u/h" ("string"), "\r") -> (w2876:string)
                    n1808 = VISA Write(VISA resource name=w2871, write buffer=w2876) -> (VISA resource name out=w2874:refnum<visa-resource-name>)  [unwired: 1 in, 2 out]
                    n1809 = Concatenate Strings("irun" ("string"), "\r") -> (w2880:string)
                    n1810 = VISA Write(VISA resource name=w2874, write buffer=w2880) -> ()  [unwired: 1 in, 3 out]
                  }
                }
                n1811 = local read "Save Event Log?"() -> (w2849:bool)
                n1812 = local read "Saving..."() -> (w2850:bool)
                n1813 = And(x=w2850, y=w2849) -> (x .and. y?=w2848:bool)
                n1814 = case shown="True" w2848 {
                  tunnel: w2851 -> [_ w2859]
                  frame False {
                  }
                  frame True {
                    n1815 = local read "Normal Flow Rate (ul/h) P3"() -> (w2853:dbl)
                    n1816 = Number To Decimal String(number=w2853) -> (decimal integer string=w2855:string)  [unwired: 1 in]
                    n1817 = Concatenate Strings("on, flow rate", w2855) -> (w2854:string)
                    n1818 = local read "log file ref"() -> (w2858:refnum<file>)
                    n1819 = Select(t=w2854, s=w2859, f="off") -> (s? t:f=w2860:string)
                    n1820 = local read "Time (s)"() -> (w2857:dbl)
                    n1821 = Concatenate Strings("pump 3 ", w2860) -> (w2862:string)
                    n1822 = call "write to event log.vi"("log file ref"=w2858, "time"=w2857, "input string"=w2862) -> ()  [unwired: 8 in]
                  }
                }
              }
            }
          }
          frame Enabled {
          }
        }
      }
      event "Inject Pump 2": Value Change {
        n1823 = event-data() -> ()  [unwired: 7 out]
        n1824 = local read "Pump write delay (ms)"() -> (w2887:dbl)
        n1825 = local read "Chemyx Syringe Pump Serial Port"() -> (w2886:refnum<visa-resource-name>)
        n1826 = flat-sequence {
          tunnel: w2886 -> [w2911]
          tunnel: w2887 -> [w2907]
          tunnel: "Inject Pump 2" -> [_]
          tunnel: w2887 -> [w2913]
          tunnel: w2886 -> [w2914]
          frame #0 {
            n1827 = local read "All Pump Parameters"() -> (w2906:T14)
            n1828 = Multiply(x=60.0, y="Flush Center Ch Rate (ul/m)") -> (x*y=w2903:dbl)
            n1829 = Unbundle By Name(w2906) -> ("Pump 2"=w2912:T58)
            n1830 = call "Set pump parameters.vi"("Pump write delay (ms)"=w2907, "Volume (uL)"="Flush Center Ch Volume (uL)", "Rate (uL/h)"=w2903, "Units"=3.0, "Pump #"=2.0, "Pump Parameters In"=w2912, "VISA resource name"=w2911) -> ("Pump Parameters Out"=w2905:T58)  [unwired: 3 in]
            n1831 = Bundle By Name(cluster=w2906, "Pump 2"=w2905) -> (w2904:T14)
            n1832 = local write "All Pump Parameters"(w2904) -> ()
            n1833 = Add(x="Flush Center Ch Volume (uL)", y="Total Volume\nFlushed (uL)") -> (x+y=w2900:dbl)
            n1834 = local write "Total Volume\nFlushed (uL)"(w2900) -> ()
          }
          frame #1 {
            n1835 = Wait (ms)(milliseconds to wait=w2913) -> ()  [unwired: 1 out]
          }
          frame #2 {
            n1836 = call "Write to pump.vi"("string"="start", "VISA resource name"=w2914) -> ()  [unwired: 1 out]
          }
        }
        n1837 = local read "Save Event Log?"() -> (w2885:bool)
        n1838 = local read "Saving..."() -> (w2884:bool)
        n1839 = And(x=w2885, y=w2884) -> (x .and. y?=w2883:bool)
        n1840 = case shown="True" w2883 {
          tunnel: "Inject Pump 2" -> [_ w2894]
          frame False {
          }
          frame True {
            n1841 = local read "Flow rate (uL/h)"() -> (w2888:dbl)
            n1842 = Number To Decimal String(number=w2888) -> (decimal integer string=w2890:string)  [unwired: 1 in]
            n1843 = Concatenate Strings("on, flow rate", w2890) -> (w2889:string)
            n1844 = Select(t=w2889, s=w2894, f="off") -> (s? t:f=w2898:string)
            n1845 = local read "Time (s)"() -> (w2892:dbl)
            n1846 = local read "log file ref"() -> (w2893:refnum<file>)
            n1847 = Concatenate Strings("pump 2 ", w2898) -> (w2896:string)
            n1848 = call "write to event log.vi"("log file ref"=w2893, "time"=w2892, "input string"=w2896) -> ()  [unwired: 8 in]
          }
        }
      }
      event "Sample Channel\nFlow": Value Change {
        n1849 = event-data() -> ()  [unwired: 7 out]
        n1850 = disable-structure shown="Disabled" {
          disable-tunnel: w2916 -> [w2923 _]
          frame Disabled {
            n1851 = Select(t="irun" ("string"), s="Sample Channel\nFlow", f="stop" ("string")) -> (s? t:f=w2918:string)
            n1852 = Concatenate Strings(w2918, "\r") -> (w2921:string)
            n1853 = VISA Write(VISA resource name=w2923, write buffer=w2921) -> ()  [unwired: 1 in, 3 out]
          }
          frame Enabled {
          }
        }
      }
      event "Start Flow": Value Change {
        n1854 = event-data() -> ()  [unwired: 7 out]
        n1855 = disable-structure shown="Disabled" {
          disable-tunnel: w2924 -> [w2925 _]
          frame Disabled {
            n1856 = local write "Sample Channel\nFlow"(TRUE ("Sample Channel\nFlow")) -> ()
            n1857 = local write "Start Flow"(FALSE ("Start Flow")) -> ()